vi "15-12-13 UHR-Fleezers Control (host) - 15.2.1UCB Darwin.vi"() -> ()   [LabVIEW 2014] (continued)
                n2143 = Transpose 2D Array(2D array=w3211) -> (transposed array=w3217:u32[][])
                n2144 = Select(t=w3217, s="Flip Y (or X)", f=w3211) -> (s? t:f=w3216:u32[][])
                n2145 = call "DMR_ImageRequestUnlock.vi"("request number IN"=w3232, "driver handle IN"=w3233) -> ("driver handle OUT"=w3238:i32)  [unwired: 1 in, 2 out]
                n2146 = for {
                  tunnel: w3216 -> [w3275] mode=indexing
                  tunnel: [w3274] -> w3214 mode=indexing
                  n2147 = Reverse 1D Array(array=w3275) -> (reversed array=w3274:u32[])
                }
                n2148 = call "DMR_ImageRequestSingle.vi"("request control IN"=0, "driver handle IN"=w3238) -> ("driver handle OUT"=w3236:i32)  [unwired: 3 out]
                n2149 = Transpose 2D Array(2D array=w3214) -> (transposed array=w3215:u32[][])
                n2150 = Select(t=w3215, s="Flip Y (or X)", f=w3214) -> (s? t:f=w3212:u32[][])
                n2151 = Select(t=w3212, s="Flip Image", f=w3211) -> (s? t:f=w3209:u32[][])
                n2152 = case shown="True" "Averaging" {
                  tunnel: w3209 -> [w3286 w3291]
                  tunnel: [w3286 w3290] -> w3223
                  tunnel: w3225 -> [_ w3288]
                  frame False {
                  }
                  frame True {
                    (unwired) 1
                    w3296 = 1
                    n2153 = feedback #2(w3288) -> (w3287:u32[][])
                    n2154 = Add(x=w3291, y=w3287) -> (x+y=w3292:u32[][])
                    n2155 = Select(t=w3288, s="Reset Averaging", f=w3292) -> (s? t:f=w3294:u32[][])
                    n2156 = feedback-in #2(w3294) -> ()
                    n2157 = feedback #3(w3296) -> (w3289:i32)
                    n2158 = Divide(x=w3292, y=w3289) -> (x/y=w3293:dbl[][])
                    n2159 = Increment(x=w3289) -> (x+1=w3297:i32)
                    n2160 = To Unsigned Long Integer(number=w3293) -> (unsigned 32bit integer=w3290:u32[][])
                    n2161 = Select(t=w3296, s="Reset Averaging", f=w3297) -> (s? t:f=w3295:i32)
                    n2162 = feedback-in #3(w3295) -> ()
                  }
                }
                n2163 = case shown="True" "Zoom video window" {
                  tunnel: w3223 -> [_ w3254]
                  tunnel: w3219 -> [_ w3253]
                  frame False {
                  }
                  frame True {
                    n2164 = To Double Precision Float(number=w3254) -> (double precision float=w3251:dbl[][])
                    n2165 = In Range and Coerce(upper limit="Intensity Upper", x=w3251, lower limit="Intensity Lower") -> (coerced(x)=w3250:dbl[][])  [unwired: 1 out]
                    n2166 = Subtract(x="Intensity Upper", y="Intensity Lower") -> (x-y=w3247:dbl)
                    n2167 = Subtract(x=w3250, y="Intensity Lower") -> (x-y=w3248:dbl[][])
                    n2168 = Divide(x=w3248, y=w3247) -> (x/y=w3249:dbl[][])
                    n2169 = Multiply(x=255.0, y=w3249) -> (x*y=w3245:dbl[][])
                    n2170 = To Unsigned Byte Integer(number=w3245) -> (unsigned 8bit integer=w3252:u8[][])
                    n2171 = call "IMAQ ArrayToImage"("Image Pixels (U8)"=w3252, "Image"=w3253) -> ("Image Out"=w3241:T2)  [unwired: 4 in, 5 out]
                    n2172 = First Call?() -> (First Call?: T/F=w3242:bool)
                    n2173 = case shown="True" w3242 {
                      tunnel: w3241 -> [w3255 w3266]
                      frame False {
                        n2174 = flat-sequence {
                          tunnel: w3255 -> [w3261]
                          frame #0 {
                            w3258 = FALSE ("Get/Set Status? (Set)")
                            w3257 = 0 ("Window Number (0...15)")
                            n2175 = call "IMAQ WindSize"("Get/Set Status? (Set)"=w3258, "Window Number"=w3257) -> ("Width & Height out"=→"Window Size":cluster{"Width":i32, "Height":i32})  [unwired: 4 in, 2 out]
                            n2176 = call "IMAQ WindMove"("Window Number (0...15)"=w3257, "Get/Set Status? (Set)"=w3258) -> ("Coordinates (screen)"=→"Window Position":cluster{"X Position":i32, "Y Position":i32})  [unwired: 3 in, 1 out]
                            n2177 = call "IMAQ WindDraw"("Resize to Image Size? (Y)"=FALSE, "Window Number (0...15)"=w3257, "Image"=w3261) -> ()  [unwired: 7 in, 2 out]
                          }
                          frame #1 {
                            n2178 = call "IMAQ WindZoom 2"("Center Point"="Center Point", "Zoom to Fit? (False)"=FALSE, "Zoom Factor"="Zoom Factor") -> ()  [unwired: 5 in, 4 out]
                          }
                        }
                      }
                      frame True {
                        n2179 = flat-sequence {
                          tunnel: w3266 -> [w3269]
                          tunnel: [w3267] -> w3265
                          tunnel: w3265 -> [w3271]
                          frame #0 {
                            w3268 = TRUE ("Resize to Image Size? (Y)")
                            w3267 = 0 ("Window Number (0...15)")
                            n2180 = call "IMAQ WindNonTearing"("Window Number"=w3267, "NonTearing? (True)"=w3268) -> ()  [unwired: 8 in, 2 out]
                            n2181 = call "IMAQ WindDraw"("Resize to Image Size? (Y)"=w3268, "Window Number (0...15)"=w3267, "Image"=w3269) -> ()  [unwired: 7 in, 2 out]
                          }
                          frame #1 {
                            n2182 = call "IMAQ WindSize"("Scrollbars? (N)"=FALSE, "Width & Height"="Initial Window Size", "Window Number"=w3271) -> ()  [unwired: 3 in, 3 out]
                            n2183 = call "IMAQ WindMove"("Window Number (0...15)"=w3271, "Coordinates (screen)"="Initial Window Position") -> ()  [unwired: 3 in, 2 out]
                          }
                        }
                      }
                    }
                  }
                }
                n2184 = To Unsigned Byte Integer(number=w3223) -> (unsigned 8bit integer=w3221:u8[][])
                n2185 = call "IMAQ ArrayToImage"("Image Pixels (U8)"=w3221, "Image"=w3222) -> ("Image Out"=w3220:T2)  [unwired: 4 in, 5 out]
                "Primary Video Display" <- w3220
                n2186 = Not(x="Close Video File") -> (.not. x?=w3207:bool)
                n2187 = And(x="Save Video", y=w3207) -> (x .and. y?=w3204:bool)
                n2188 = case shown="True" "Save Image" {
                  tunnel: w3221 -> [_ w3300]
                  tunnel: w3218 -> [_ w3299]
                  frame False {
                  }
                  frame True {
                    n2189 = call <vilib>:"Flatten Pixmap.vi"("colors"=w3299, "8-bit pixmap"=w3300) -> ("image data"=w3306:T41)  [unwired: 4 in, 5 out]
                    n2190 = call "Create new save file.vi"("Insert"="video_frame_" ("string"), "Ext"=".bmp" ("string"), "Index In"="Image Index") -> ("Path Out"=w3302:path, "Index Out"=w3307:dbl)
                    n2191 = Increment(x=w3307) -> (x+1=w3301:dbl)
                    n2192 = local write "Image Index"(w3301) -> ()
                    n2193 = call <vilib>:"Write BMP File.vi"("image data"=w3306, "path to BMP file"=w3302) -> ()  [unwired: 1 in, 9 out]
                  }
                }
                n2194 = case shown="True" w3204 {
                  tunnel: w3205 -> [w3277 w3282]
                  tunnel: w3220 -> [_ w3281]
                  tunnel: "Close Video File" -> [w3276 _]
                  frame False {
                    n2195 = case shown="True" w3276 {
                      tunnel: w3277 -> [_ w3278]
                      frame False {
                      }
                      frame True {
                        w3279 = FALSE ("Save Video")
                        n2196 = call "IMAQ AVI2 Close"("AVI Refnum"=w3278) -> ()  [unwired: 10 in, 1 out]
                        n2197 = local write "File open?"(w3279) -> ()
                        n2198 = local write "Save Video"(w3279) -> ()
                      }
                    }
                  }
                  frame True {
                    n2199 = local read "File open?"() -> (w3280:bool)
                    n2200 = case shown="True" w3280 {
                      tunnel: w3282 -> [_ w3285]
                      tunnel: w3281 -> [_ w3284]
                      frame False {
                        n2201 = local write "New Video File"(TRUE ("New Video File")) -> ()
                      }
                      frame True {
                        n2202 = call "IMAQ AVI2 Write Frame"("Image"=w3284, "AVI Refnum"=w3285) -> ()  [unwired: 7 in, 3 out]
                      }
                    }
                  }
                }
              }
            }
            n2203 = node-c288(w3167, "Deadline (ms)") -> ()  [unwired: 1 out]
          }
          n2204 = node-c288(w3147) -> ()  [unwired: 1 out]
          n2205 = call "DMR_CloseDevice.vi"("driver handle IN"=w3152) -> ()  [unwired: 1 in, 4 out]
        }
        frame #4 {
          n2206 = call "DMR_Close.vi"() -> ()  [unwired: 1 out]
        }
      }
    }
    frame Enabled {
    }
  }
  n2207 = node-c288(3 ("Processor")) -> (w57:T27)  [unwired: 3 out]
  n2208 = timed-loop "Oscillate Trap/AOM (fishing, conjugate plane alignment)" {
    tunnel: [w3314] -> w62
    timing: w57 -> [_]
    timing-out: [_] -> w56
    tunnel: w15 -> [w3313]
    tunnel: w3 -> [w3312]
    stop <- w3314 stop-if-true
    n2209 = node-c288() -> ()  [unwired: 2 out]
    n2210 = event shown="[2] \"Start assembly line\": Value Change" {
      selector: _ -> [_ _ _ _]
      dyn-events: _ -> [_ _ _ _]
      timeout: _ -> [_ _ _ _]
      tunnel: [FALSE ("Stop All") _ _ w3985] -> w3314
      tunnel: w3313 -> [w3317 _ _ _]
      tunnel: w3312 -> [_ _ w3922 _]
      event "Oscillate Set 1", "Fish for Tether": Value Change {
        n2211 = event-data() -> ()  [unwired: 6 out]
        n2212 = local read "Oscillate Set 1"() -> (w3321:bool)
        n2213 = Or(x=w3321, y="Fish for Tether") -> (x .or. y?=w3319:bool)
        n2214 = case shown="True" w3319 {
          tunnel: "Fish for Tether" -> [_ w3324]
          tunnel: w3317 -> [_ w3322]
          frame False {
          }
          frame True {
            n2215 = case shown="True" w3324 {
              selector: w3324 -> [w3327 w3333]
              tunnel: [w3327 w3333] -> w3323
              frame False {
              }
              frame True {
                n2216 = local write "Scan axis 2"(TRUE) -> ()
                n2217 = local write "Tether"(FALSE ("Tether")) -> ()
                n2218 = local read "Flow ON during cal?"() -> (w3328:bool)
                n2219 = property on="Trap Delta (MHz)" class="DigNum (strict)"("Val(Sgnl)"="Furthest Delta (MHz)") -> ()  [unwired: 2 in, 2 out]
                n2220 = Or(x="Flow ON during \nfishing?", y=w3328) -> (x .or. y?=w3329:bool)
                n2221 = Wait (ms)(milliseconds to wait=u32 500) -> ()  [unwired: 1 out]
                n2222 = property on="Sample Channel\nFlow" class="Bool (strict)"("Val(Sgnl)"=w3329) -> ()  [unwired: 2 in, 2 out]
              }
            }
            n2223 = node-c288() -> (w3326:T27)  [unwired: 1 in, 3 out]
            n2224 = timed-loop "Oscillate AOD" {
              timing: w3326 -> [_]
              timing-out: [_] -> w3325
              tunnel: w3323 -> [w3337]
              tunnel: w3322 -> [w3336]
              i -> [w3345]
              stop <- w3343 stop-if-true
              n2225 = node-c288() -> (w3344:i64)  [unwired: 1 out]
              n2226 = flat-sequence {
                tunnel: w3345 -> [w3372]
                tunnel: w3344 -> [w3371]
                tunnel: w3337 -> [w3355]
                tunnel: [w3355] -> w3342
                tunnel: [w3354] -> w3341
                tunnel: [w3353] -> w3340
                tunnel: [w3350] -> w3338
                tunnel: w3336 -> [w3346]
                tunnel: w3342 -> [w3419]
                tunnel: w3341 -> [w3417]
                tunnel: w3340 -> [w3416]
                tunnel: [w3415] -> w3339
                tunnel: w3338 -> [w3414]
                tunnel: [w3491] -> w3343
                tunnel: w3339 -> [w3490]
                frame #0 {
                  # "w (rad/s)"
                  # "t (s)"
                  n2227 = Divide(x=w3371, y=i64 1000) -> (x/y=w3347:dbl)
                  n2228 = local read "BD 1 Frequency 2 (MHz)"() -> (w3349:dbl)
                  n2229 = Multiply(x="Osc. freq. (Hz)", y=6.283185307179586) -> (x*y=w3369:dbl)
                  n2230 = Multiply(x=w3347, y=w3372) -> (x*y=w3368:dbl)
                  n2231 = Multiply(x=w3369, y=w3368) -> (x*y=w3352:dbl)
                  n2232 = local read "BD 1 Frequency 1 (MHz)"() -> (w3357:dbl)
                  n2233 = case shown="True" w3355 {
                    tunnel: w3352 -> [w3378 w3397]
                    tunnel: w3357 -> [_ w3405]
                    tunnel: w3349 -> [_ w3406]
                    tunnel: [w3375 w3401] -> w3348
                    tunnel: [FALSE w3379] -> w3353
                    tunnel: [0.0 w3393] -> w3350
                    frame False {
                      n2234 = Sine(x=w3378) -> (sin(x)=w3376:dbl)
                      n2235 = Multiply(x=w3376, y="Osc. amp. (MHz)") -> (x*y=w3375:dbl)
                    }
                    frame True {
                      # "trap position goes from 0 to 1 (0 is when it is furthest away, 1 is when closest)\nso we want to test for tether only when farther away, or x < 1"
                      # "quit if taking too long"
                      # "oscillate the trap"
                      # "Test for tether"
                      n2236 = local read "Vec Mean of T1 T2"() -> (w3382:dbl[])
                      "Trigger Signal" <- w3382
                      n2237 = Cosine(x=w3397) -> (cos(x)=w3409:dbl)
                      n2238 = Subtract(x=w3406, y=w3405) -> (x-y=w3404:dbl)
                      n2239 = Decrement(x=w3409) -> (x-1=w3408:dbl)
                      n2240 = Subtract(x=w3404, y="Closest Delta (MHz)") -> (x-y=w3402:dbl)
                      n2241 = Divide(x=w3408, y=-2.0) -> (x/y=w3392:dbl)
                      n2242 = Greater?(x=w3382, y="Stop F (pN)") -> (0:w3399:bool[])
                      n2243 = Multiply(x=w3392, y=w3402) -> (x*y=w3401:dbl)
                      n2244 = Less?(x=w3392, y="Fish mask thresh") -> (x < y?=w3391:bool)
                      n2245 = Boolean To (0,1)(Boolean=w3391) -> (0, 1=w3389:i16)
                      n2246 = Multiply(x=w3389, y=w3382) -> (x*y=w3388:dbl[])
                      n2247 = Divide(x=w3397, y=6.283185307179586) -> (x/y=w3396:dbl)
                      n2248 = Round Toward +Infinity(x=w3396) -> (ceil(x): smallest int >= x=w3393:dbl)
                      "Attempts" <- w3393
                      n2249 = Greater?(x=w3388, y="Stop F (pN) (mask)") -> (0:w3386:bool[])
                      n2250 = Or Array Elements(Boolean array=w3399) -> (logical OR=w3384:bool)
                      n2251 = Or Array Elements(Boolean array=w3386) -> (logical OR=w3383:bool)
                      n2252 = Greater?(x=w3393, y="Attempt Limit") -> (0:w3395:bool)
                      n2253 = case shown="True" w3395 {
                        frame False {
                        }
                        frame True {
                          n2254 = local write "Fish for Tether"(FALSE ("Fish for Tether")) -> ()
                          n2255 = call <vilib>:"Beep.vi"() -> ()  [unwired: 3 in, 9 out]
                          n2256 = local read "Messages"() -> (w3411:string)
                          n2257 = call "Update messages.vi"("Message to add"="Tether fishing timeout." ("Messages"), "Old message string"=w3411) -> ("New message string"=→"Messages":string)
                        }
                      }
                      n2258 = Select(t=w3384, s="Normal (on) or masked test (off)", f=w3383) -> (s? t:f=w3381:bool)
                      n2259 = And(x="Stop Fishing When Tether", y=w3381) -> (x .and. y?=w3379:bool)
                    }
                  }
                  n2260 = local read "BD 2 Frequency 1 (MHz)"() -> (w3356:dbl)
                  n2261 = Select(t=w3357, s="Scan axis 2", f=w3356) -> (s? t:f=w3360:dbl)
                  n2262 = Add(x=w3348, y=w3360) -> (x+y=w3354:dbl)
                  n2263 = Select(t=w3354, s="Scan axis 2", f=w3357) -> (s? t:f=w3363:dbl)
                  n2264 = Select(t=w3356, s="Scan axis 2", f=w3354) -> (s? t:f=w3362:dbl)
                  n2265 = local read "BD 2 Frequency 2 (MHz)"() -> (w3365:dbl)
                  n2266 = local read "BD 2 Frequency 3 (MHz)"() -> (w3364:dbl)
                  n2267 = local read "Y RF Frequency Limits (MHz)"() -> (w3358:T18)
                  n2268 = local read "X RF Frequency Limits (MHz)"() -> (w3359:T18)
                  n2269 = local read "BD 1 Frequency 3 (MHz)"() -> (w3366:dbl)
                  n2270 = call "set RF board frequency - interlace.vi"("Board 2 Frequency Limits"=w3358, "Board 1 Frequency Limits"=w3359, "FPGA VI Reference In"=w3346, "Board 2 Frequency 3 (MHz)"=w3364, "Board 1 Frequency 3 (MHz)"=w3366, "Board 2 Frequency 2 (MHz)"=w3365, "Board 2 Frequency 1 (MHz)"=w3362, "Board 1 Frequency 2 (MHz)"=w3349, "Board 1 Frequency 1  (MHz)"=w3363) -> ()  [unwired: 1 in, 2 out]
                }
                frame #1 {
                  n2271 = And(x=w3419, y=w3416) -> (x .and. y?=w3418:bool)
                  n2272 = case "Only if were fishing and now formed tether" shown="True" w3418 {
                    tunnel: w3417 -> [w3421 w3436]
                    tunnel: [w3420 w3435] -> w3415
                    tunnel: w3414 -> [_ w3431]
                    frame False {
                      n2273 = local read "Fish for Tether"() -> (w3420:bool)
                      n2274 = case shown="False" w3420 {
                        tunnel: w3421 -> [w3422 _]
                        frame False {
                          n2275 = property on="BD 1 Frequency 1 (MHz)" class="DigNum (strict)"("Val(Sgnl)"=w3422) -> ()  [unwired: 2 in, 2 out]
                        }
                        frame True {
                        }
                      }
                    }
                    frame True {
                      w3435 = FALSE ("Fish for Tether")
                      n2276 = call <vilib>:"Beep.vi"() -> ()  [unwired: 3 in, 9 out]
                      n2277 = Number To Decimal String(number=w3431, width (-)=i16 1) -> (decimal integer string=w3429:string)
                      n2278 = Concatenate Strings("Formed tether in ", w3429, " attempt(s)." ("string")) -> (w3426:string)
                      n2279 = local read "Messages"() -> (w3433:string)
                      n2280 = local write "Fish for Tether"(w3435) -> ()
                      n2281 = call "Update messages.vi"("Message to add"=w3426, "Old message string"=w3433) -> ("New message string"=w3432:string)
                      n2282 = local write "Messages"(w3432) -> ()
                      n2283 = Get Date/Time In Seconds() -> (seconds since 1Jan1904=→"Time tether formed":timestamp)
                      n2284 = local read "Flow ON during cal?"() -> (w3423:bool)
                      n2285 = property on="Sample Channel\nFlow" class="Bool (strict)"("Val(Sgnl)"=w3423) -> (error out=w3424:errorcluster)  [unwired: 2 in, 1 out]
                      n2286 = case shown="\"2\", \"3\", \"4\", \"5\", \"6\"" "Then..." {
                        selector: "Then..." -> [_ w3439]
                        tunnel: w3436 -> [w3438 _]
                        tunnel: w3424 -> [_ _]
                        frame "1", Default {
                          n2287 = property on="BD 1 Frequency 1 (MHz)" class="DigNum (strict)"("Val(Sgnl)"=w3438) -> ()  [unwired: 2 in, 2 out]
                        }
                        frame "2", "3", "4", "5", "6" {
                          n2288 = flat-sequence {
                            tunnel: w3439 -> [w3441]
                            frame #0 {
                              n2289 = property on="Trap Delta (MHz)" class="DigNum (strict)"("Val(Sgnl)"="Move to Delta 1 (MHz)") -> ()  [unwired: 2 in, 2 out]
                            }
                            frame #1 {
                              n2290 = case shown="\"5\", \"6\"" w3441 {
                                selector: w3441 -> [w3444 w3454 _]
                                frame "3", "4" {
                                n2291 = flat-sequence {
                                tunnel: w3444 -> [w3445]
                                tunnel: [w3445] -> w3442
                                tunnel: [w3447] -> w3443
                                tunnel: w3442 -> [w3447]
                                tunnel: w3443 -> [w3451]
                                frame #0 {
                                n2292 = property on="Green Laser ON" class="Bool (strict)"("Val(Sgnl)"=TRUE ("Value (Signaling)")) -> ()  [unwired: 2 in, 2 out]
                                }
                                frame #1 {
                                n2293 = Multiply(x="Wait Before Save (s)", y=u32 1000 ("x")) -> (x*y=w3449:u32)
                                n2294 = Wait (ms)(milliseconds to wait=w3449) -> ()  [unwired: 1 out]
                                }
                                frame #2 {
                                n2295 = property on="Start Saving" class="Bool (strict)"("Value"=TRUE ("Start Saving")) -> ()  [unwired: 2 in, 2 out]
                                n2296 = case shown="\"4\"" w3451 {
                                frame Default {
                                }
                                frame "4" {
                                n2297 = property on="Fl. Triggered..." class="Bool (strict)"("Val(Sgnl)"=TRUE ("Value (Signaling)")) -> ()  [unwired: 2 in, 2 out]
                                }
                                }
                                }
                                }
                                }
                                frame "5", "6" {
                                n2298 = stacked-sequence {
                                tunnel: w3454 -> [_ _ _ _ _ _ w3466]
                                frame #0 {
                                n2299 = Replace Array Subset(array=u32[] [0] ("Index Values"), new element="Raster Set Upon Tether", index=0) -> (w3455:u32[])
                                n2300 = property on="Saved AOD Raster Scan Parameter Sets" class="Arr (strict)"("Index Values"=w3455) -> ()  [unwired: 2 in, 2 out]
                                }
                                frame #1 {
                                n2301 = Wait (ms)(milliseconds to wait=u32 500) -> ()  [unwired: 1 out]
                                }
                                frame #2 {
                                n2302 = property on="Load parameters" class="Bool (strict)"("Val(Sgnl)"=TRUE ("Value (Signaling)")) -> ()  [unwired: 2 in, 2 out]
                                n2303 = case shown="True" "Green ON During Raster" {
                                frame False {
                                }
                                frame True {
                                n2304 = property on="Green Laser ON" class="Bool (strict)"("Val(Sgnl)"=TRUE ("Value (Signaling)")) -> ()  [unwired: 2 in, 2 out]
                                }
                                }
                                }
                                frame #3 {
                                n2305 = Wait (ms)(milliseconds to wait=u32 500) -> ()  [unwired: 1 out]
                                }
                                frame #4 {
                                n2306 = property on="Trap Raster Scan" class="Bool (strict)"("Val(Sgnl)"=TRUE ("Value (Signaling)")) -> ()  [unwired: 2 in, 2 out]
                                }
                                frame #5 {
                                n2307 = Wait (ms)(milliseconds to wait=u32 2000) -> ()  [unwired: 1 out]
                                }
                                frame #6 {
                                n2308 = flat-sequence {
                                tunnel: w3466 -> [w3473]
                                frame #0 {
                                n2309 = while {
                                stop <- w3469 stop-if-true
                                n2310 = local read "Raster Scanning..."() -> (w3468:bool)
                                n2311 = local read "Saving..."() -> (w3471:bool)
                                n2312 = Wait (ms)(milliseconds to wait=u32 100) -> ()  [unwired: 1 out]
                                n2313 = Not(x=w3471) -> (.not. x?=w3470:bool)
                                n2314 = Not(x=w3468) -> (.not. x?=w3467:bool)
                                n2315 = And(x=w3470, y=w3467) -> (x .and. y?=w3469:bool)
                                }
                                }
                                frame #1 {
                                n2316 = local read "Tether"() -> (w3474:bool)
                                n2317 = case shown="True" w3474 {
                                tunnel: w3473 -> [_ w3476]
                                frame False {
                                n2318 = property on="Fish for Tether" class="Bool (strict)"("Val(Sgnl)"="Fish again after \nraster break?") -> ()  [unwired: 2 in, 2 out]
                                }
                                frame True {
                                n2319 = stacked-sequence {
                                tunnel: w3476 -> [_ w3480 _ _]
                                frame #0 {
                                n2320 = property on="Trap Delta (MHz)" class="DigNum (strict)"("Val(Sgnl)"="Move to Delta 2 (MHz)") -> ()  [unwired: 2 in, 2 out]
                                n2321 = case shown="True" "Flow ON after\ntether testing?" {
                                frame False {
                                }
                                frame True {
                                n2322 = property on="Sample Channel\nFlow" class="Bool (strict)"("Val(Sgnl)"=TRUE ("Value (Signaling)")) -> ()  [unwired: 2 in, 2 out]
                                }
                                }
                                }
                                frame #1 {
                                n2323 = flat-sequence {
                                tunnel: w3480 -> [w3482]
                                frame #0 {
                                n2324 = Wait (ms)(milliseconds to wait=u32 500) -> ()  [unwired: 1 out]
                                }
                                frame #1 {
                                n2325 = case shown="\"6\"" w3482 {
                                frame Default {
                                }
                                frame "6" {
                                n2326 = property on="Green Laser ON" class="Bool (strict)"("Val(Sgnl)"=TRUE ("Green Laser ON/Interlacing")) -> ()  [unwired: 2 in, 2 out]
                                }
                                }
                                }
                                frame #2 {
                                n2327 = Wait (ms)(milliseconds to wait=u32 500) -> ()  [unwired: 1 out]
                                }
                                frame #3 {
                                n2328 = local write "Start Saving"("Save at end (5, 6)") -> ()
                                }
                                }
                                }
                                frame #2 {
                                n2329 = local read "Bead Sep. Int. Time (s)"() -> (w3488:dbl)
                                n2330 = Multiply(x=w3488, y=1000.0) -> (x*y=w3487:dbl)
                                n2331 = Wait (ms)(milliseconds to wait=w3487) -> ()  [unwired: 1 out]
                                }
                                frame #3 {
                                n2332 = property on="Remove Offset" class="Bool (strict)"("Val(Sgnl)"=TRUE ("Value (Signaling)")) -> ()  [unwired: 2 in, 2 out]
                                }
                                }
                                }
                                }
                                }
                                }
                                }
                                }
                                }
                                frame "2", Default {
                                }
                              }
                            }
                          }
                        }
                      }
                      "Tether" <- "Tether Alarm?"
                    }
                  }
                }
                frame #2 {
                  n2333 = local read "Oscillate Set 1"() -> (w3495:bool)
                  n2334 = local read "Stop All"() -> (w3493:bool)
                  n2335 = Or(x=w3495, y=w3490) -> (x .or. y?=w3492:bool)
                  n2336 = Not(x=w3492) -> (.not. x?=w3494:bool)
                  n2337 = Compound Arithmetic op=OR(w3493, w3494) -> (w3491:bool)
                }
              }
              n2338 = node-c288() -> ()  [unwired: 2 out]
            }
            n2339 = node-c288(w3325) -> ()  [unwired: 1 out]
          }
        }
      }
      event "Fl. Triggered...": Value Change {
        n2340 = event-data() -> ()  [unwired: 7 out]
        n2341 = case shown="True" "Fl. Triggered..." {
          frame False {
          }
          frame True {
            n2342 = node-c288() -> (w3506:T27)  [unwired: 4 out]
            n2343 = timed-loop {
              timing: w3506 -> [_]
              timing-out: [_] -> w3505
              tunnel: "Action" -> [w3514]
              shift-right: [w3511] -> _
              shift-left: u8 255 -> [w3513]
              shift-right: [w3508] -> _
              shift-left: 255 -> [w3510]
              stop <- w3507 stop-if-true
              # "Reset confocal spot"
              n2344 = node-c288() -> ()  [unwired: 2 out]
              n2345 = flat-sequence {
                tunnel: w3514 -> [w3534]
                tunnel: w3513 -> [w3533]
                tunnel: [w3532] -> w3512
                tunnel: w3510 -> [w3519]
                tunnel: [w3518] -> w3509
                tunnel: [w3913] -> w3507
                tunnel: w3512 -> [w3912]
                tunnel: [w3912] -> w3511
                tunnel: [w3911] -> w3508
                tunnel: w3509 -> [w3911]
                frame #0 {
                  n2346 = local read "Delta Fl. 2"() -> (w3531:dbl)
                  n2347 = local read "Delta Fl. 1"() -> (w3526:dbl)
                  n2348 = Multiply(x="Fl. Delta Thresh. (kHz)", y=1000.0) -> (x*y=w3521:dbl)
                  n2349 = Select(t=w3526, s="APD to Watch", f=w3531) -> (s? t:f=w3522:dbl)
                  n2350 = Greater?(x=w3522, y=w3521) -> (0:w3527:bool)
                  n2351 = Or(x="Force Yank", y=w3527) -> (x .or. y?=w3525:bool)
                  n2352 = And(x=w3525, y="Yank when?") -> (x .and. y?=w3523:bool)
                  n2353 = case shown="False" w3523 {
                    tunnel: w3534 -> [w3537 w3738]
                    tunnel: w3533 -> [w3539 w3734]
                    tunnel: [w3539 w3732] -> w3532
                    tunnel: w3522 -> [w3545 _]
                    tunnel: w3521 -> [w3544 _]
                    tunnel: "Force Yank" -> [w3542 _]
                    tunnel: w3519 -> [w3541 w3731]
                    tunnel: [w3540 w3731] -> w3518
                    frame False {
                      n2354 = Negate(x=w3544) -> (-x=w3536:dbl)
                      n2355 = local write "Fl. High"(TRUE ("Fl. High")) -> ()
                      n2356 = Less?(x=w3545, y=w3536) -> (x < y?=w3543:bool)
                      n2357 = Or(x=w3542, y=w3543) -> (x .or. y?=w3538:bool)
                      n2358 = case shown="True" w3538 {
                        tunnel: w3541 -> [w3546 w3556]
                        tunnel: [w3546 w3555] -> w3540
                        tunnel: w3537 -> [_ w3554]
                        frame False {
                        }
                        frame True {
                          n2359 = flat-sequence {
                            tunnel: w3556 -> [w3562]
                            tunnel: w3554 -> [w3559]
                            tunnel: [w3561] -> w3553
                            tunnel: [w3560] -> w3552
                            tunnel: [w3559] -> w3551
                            tunnel: w3550 -> [w3558]
                            tunnel: [w3558] -> w3549
                            tunnel: w3548 -> [w3557]
                            tunnel: [w3557] -> w3547
                            tunnel: [w3633] -> w3555
                            tunnel: w3553 -> [w3633]
                            tunnel: w3552 -> [w3632]
                            tunnel: w3551 -> [w3631]
                            tunnel: w3549 -> [w3630]
                            tunnel: w3547 -> [w3629]
                            frame #0 {
                              n2360 = call <vilib>:"Beep.vi"() -> ()  [unwired: 12 in]
                              n2361 = local write "Waiting"(FALSE ("Waiting")) -> ()
                              n2362 = Increment(x=w3562) -> (x+1=w3561:i32)
                              n2363 = case shown="\"Image\"" w3559 {
                                tunnel: w3561 -> [_ w3567 _]
                                frame "Alarm", Default {
                                }
                                frame "Yank" {
                                n2364 = flat-sequence {
                                tunnel: w3567 -> [w3570]
                                tunnel: [w3569] -> w3566
                                tunnel: [w3568] -> w3565
                                tunnel: w3566 -> [w3580]
                                tunnel: w3565 -> [w3581]
                                frame #0 {
                                n2365 = local read "Yank Delay (s)"() -> (w3573:dbl)
                                n2366 = local read "N Array El"() -> (w3568:u8)
                                n2367 = Quotient & Remainder(x=w3570, y=w3568) -> (x-y*floor(x/y)=w3569:i32)  [unwired: 1 out]
                                n2368 = Multiply(x=w3573, y=1000.0) -> (x*y=w3571:dbl)
                                n2369 = Wait (ms)(milliseconds to wait=w3571) -> ()  [unwired: 1 out]
                                }
                                frame #1 {
                                n2370 = local read "Yank to which?"() -> (w3575:bool)
                                n2371 = local read "Random Choice"() -> (w3585:bool)
                                n2372 = local read "Yank to Trap Delta (MHz)"() -> (w3578:dbl[])
                                n2373 = local read "Yank to SP"() -> (w3579:dbl[])
                                n2374 = Random Number (0-1)() -> (number: 0 to 1=w3584:dbl)
                                n2375 = Multiply(x=w3581, y=w3584) -> (x*y=w3583:dbl)
                                n2376 = Round Toward -Infinity(1:w3583) -> (0:w3582:dbl)
                                n2377 = Select(t=w3582, s=w3585, f=w3580) -> (s? t:f=w3576:dbl)
                                n2378 = Select(t=w3578, s=w3575, f=w3579) -> (s? t:f=w3577:dbl[])
                                n2379 = Index Array(array=w3577, index=w3576) -> (element=w3574:dbl)
                                n2380 = case shown="True" w3575 {
                                tunnel: w3574 -> [w3586 w3613]
                                frame False {
                                n2381 = flat-sequence {
                                tunnel: w3586 -> [w3587]
                                frame #0 {
                                n2382 = property on="Trap Pos FB SP" class="DigNum (strict)"("Val(Sgnl)"=w3587) -> ()  [unwired: 2 in, 2 out]
                                }
                                frame #1 {
                                n2383 = Wait (ms)(milliseconds to wait=u32 700) -> ()  [unwired: 1 out]
                                }
                                frame #2 {
                                n2384 = local read "Action (%)"() -> (w3592:dbl)
                                n2385 = Absolute Value(x=w3592) -> (abs(x)=w3591:dbl)
                                n2386 = Greater?(x=w3591, y=70.0) -> (0:w3589:bool)
                                n2387 = property on="Remove Action Offset" class="Bool (strict)"("Val(Sgnl)"=w3589) -> ()  [unwired: 2 in, 2 out]
                                }
                                frame #3 {
                                n2388 = for {
                                N: 4 -> [_]
                                n2389 = flat-sequence {
                                frame #0 {
                                n2390 = Wait (ms)(milliseconds to wait=u32 500) -> ()  [unwired: 1 out]
                                }
                                frame #1 {
                                n2391 = local read "Action (%)"() -> (w3598:dbl)
                                n2392 = Absolute Value(x=w3598) -> (abs(x)=w3597:dbl)
                                n2393 = Greater?(x=w3597, y=70.0) -> (0:w3595:bool)
                                n2394 = property on="Remove Action Offset" class="Bool (strict)"("Val(Sgnl)"=w3595) -> ()  [unwired: 2 in, 2 out]
                                }
                                }
                                }
                                }
                                frame #4 {
                                n2395 = Wait (ms)(milliseconds to wait=u32 500) -> ()  [unwired: 1 out]
                                }
                                frame #5 {
                                n2396 = local read "Mean"() -> (w3606:dbl)
                                n2397 = Greater?(x=w3606, y=11.0) -> (0:w3600:bool)
                                n2398 = Not(x=w3600) -> (.not. x?=w3601:bool)
                                n2399 = And(x=w3601, y="Shift confocal") -> (x .and. y?=w3603:bool)
                                n2400 = And(x=w3600, y="Shift confocal") -> (x .and. y?=w3604:bool)
                                n2401 = case shown="True" w3604 {
                                frame False {
                                }
                                frame True {
                                n2402 = local read "Confocal Y 2 (V)"() -> (w3610:dbl)
                                n2403 = local read "Confocal X 2 (V)"() -> (w3609:dbl)
                                n2404 = property on="AO1" class="Slide (strict)"("Val(Sgnl)"=w3610) -> ()  [unwired: 2 in, 2 out]
                                n2405 = property on="AO2" class="Slide (strict)"("Val(Sgnl)"=w3609) -> ()  [unwired: 2 in, 2 out]
                                }
                                }
                                n2406 = case shown="True" w3603 {
                                frame False {
                                }
                                frame True {
                                n2407 = local read "Confocal Y 1 (V)"() -> (w3608:dbl)
                                n2408 = local read "Confocal X 1 (V)"() -> (w3607:dbl)
                                n2409 = property on="AO1" class="Slide (strict)"("Val(Sgnl)"=w3608) -> ()  [unwired: 2 in, 2 out]
                                n2410 = property on="AO2" class="Slide (strict)"("Val(Sgnl)"=w3607) -> ()  [unwired: 2 in, 2 out]
                                }
                                }
                                }
                                frame #6 {
                                n2411 = Wait (ms)(milliseconds to wait=u32 1500) -> ()  [unwired: 1 out]
                                }
                                frame #7 {
                                n2412 = property on="Rem fb disp offset" class="Bool (strict)"("Val(Sgnl)"=TRUE ("Value (Signaling)")) -> ()  [unwired: 2 in, 2 out]
                                }
                                }
                                }
                                frame True {
                                n2413 = flat-sequence {
                                tunnel: w3613 -> [w3614]
                                frame #0 {
                                n2414 = property on="Trap Delta (MHz)" class="DigNum (strict)"("Val(Sgnl)"=w3614) -> ()  [unwired: 2 in, 2 out]
                                }
                                frame #1 {
                                n2415 = Wait (ms)(milliseconds to wait=u32 500) -> ()  [unwired: 1 out]
                                }
                                frame #2 {
                                n2416 = local read "Shift confocal"() -> (w3620:bool)
                                n2417 = local read "Mean"() -> (w3622:dbl)
                                n2418 = Greater?(x=w3622, y=11.0) -> (0:w3619:bool)
                                n2419 = Not(x=w3619) -> (.not. x?=w3618:bool)
                                n2420 = And(x=w3618, y=w3620) -> (x .and. y?=w3616:bool)
                                n2421 = And(x=w3619, y=w3620) -> (x .and. y?=w3617:bool)
                                n2422 = case shown="True" w3617 {
                                frame False {
                                }
                                frame True {
                                n2423 = local read "Confocal Y 2 (V)"() -> (w3626:dbl)
                                n2424 = local read "Confocal X 2 (V)"() -> (w3625:dbl)
                                n2425 = property on="AO2" class="Slide (strict)"("Val(Sgnl)"=w3625) -> ()  [unwired: 2 in, 2 out]
                                n2426 = property on="AO1" class="Slide (strict)"("Val(Sgnl)"=w3626) -> ()  [unwired: 2 in, 2 out]
                                }
                                }
                                n2427 = case shown="True" w3616 {
                                frame False {
                                }
                                frame True {
                                n2428 = local read "Confocal X 1 (V)"() -> (w3623:dbl)
                                n2429 = local read "Confocal Y 1 (V)"() -> (w3624:dbl)
                                n2430 = property on="AO2" class="Slide (strict)"("Val(Sgnl)"=w3623) -> ()  [unwired: 2 in, 2 out]
                                n2431 = property on="AO1" class="Slide (strict)"("Val(Sgnl)"=w3624) -> ()  [unwired: 2 in, 2 out]
                                }
                                }
                                }
                                }
                                }
                                }
                                }
                                }
                                }
                                frame "Image" {
                                n2432 = property on="Confocal Image" class="Bool (strict)"("Val(Sgnl)"=TRUE ("Value (Signaling)")) -> ()  [unwired: 2 in, 2 out]
                                }
                              }
                              n2433 = local write "Fl. High"(FALSE ("Fl. High")) -> ()
                              n2434 = local read "Time (s)"() -> (w3560:dbl)
                            }
                            frame #1 {
                              n2435 = case shown="True" "Auto F Reset" {
                                tunnel: w3632 -> [_ w3637]
                                tunnel: w3631 -> [_ w3636]
                                tunnel: w3630 -> [_ w3635]
                                tunnel: w3629 -> [_ w3634]
                                frame False {
                                }
                                frame True {
                                n2436 = node-c288() -> (w3639:T27)  [unwired: 4 in]
                                n2437 = timed-loop {
                                timing: w3639 -> [_]
                                timing-out: [_] -> w3638
                                tunnel: w3637 -> [w3644]
                                tunnel: w3636 -> [w3643]
                                tunnel: w3635 -> [w3642]
                                tunnel: w3634 -> [w3641]
                                stop <- w3640 stop-if-true
                                n2438 = node-c288() -> ()  [unwired: 1 in, 1 out]
                                n2439 = local read "Fl. Delta Thresh. (kHz)"() -> (w3653:dbl)
                                n2440 = local read "APD to Watch"() -> (w3654:bool)
                                n2441 = local read "Delta Fl. 1"() -> (w3655:dbl)
                                n2442 = local read "Delta Fl. 2"() -> (w3656:dbl)
                                n2443 = local read "Fl. Triggered..."() -> (w3647:bool)
                                n2444 = local read "Stop All"() -> (w3648:bool)
                                n2445 = local read "Reset Force"() -> (w3646:bool)
                                n2446 = Multiply(x=w3653, y=1000.0) -> (x*y=w3651:dbl)
                                n2447 = Select(t=w3655, s=w3654, f=w3656) -> (s? t:f=w3650:dbl)
                                n2448 = Not(x=w3647) -> (.not. x?=w3645:bool)
                                n2449 = Greater?(x=w3650, y=w3651) -> (0:w3649:bool)
                                n2450 = Compound Arithmetic op=OR(w3649, w3648, w3645, w3646) -> (w3640:bool)
                                n2451 = case shown="True" w3640 {
                                tunnel: w3644 -> [_ w3660]
                                tunnel: w3643 -> [_ w3664]
                                tunnel: w3642 -> [_ w3663]
                                tunnel: w3641 -> [_ w3662]
                                frame False {
                                }
                                frame True {
                                n2452 = case shown="\"Yank\"" w3664 {
                                tunnel: w3663 -> [_ w3674]
                                tunnel: w3662 -> [_ w3672]
                                frame "Image", Default {
                                }
                                frame "Yank" {
                                n2453 = flat-sequence {
                                tunnel: [w3677] -> w3675
                                tunnel: w3674 -> [w3677]
                                tunnel: [w3676] -> w3673
                                tunnel: w3672 -> [w3676]
                                tunnel: w3675 -> [w3683]
                                tunnel: w3673 -> [w3681]
                                frame #0 {
                                n2454 = local read "Yank Delay (s)"() -> (w3680:dbl)
                                n2455 = Multiply(x=w3680, y=1000.0) -> (x*y=w3678:dbl)
                                n2456 = Wait (ms)(milliseconds to wait=w3678) -> ()  [unwired: 1 out]
                                }
                                frame #1 {
                                n2457 = local read "Yank to which?"() -> (w3682:bool)
                                n2458 = case shown="False" w3682 {
                                tunnel: w3683 -> [_ w3711]
                                tunnel: w3681 -> [w3684 _]
                                frame False {
                                n2459 = flat-sequence {
                                tunnel: w3684 -> [w3685]
                                frame #0 {
                                n2460 = property on="Trap Pos FB SP" class="DigNum (strict)"("Val(Sgnl)"=w3685) -> ()  [unwired: 2 in, 2 out]
                                }
                                frame #1 {
                                n2461 = Wait (ms)(milliseconds to wait=u32 700) -> ()  [unwired: 1 out]
                                }
                                frame #2 {
                                n2462 = local read "Action (%)"() -> (w3690:dbl)
                                n2463 = Absolute Value(x=w3690) -> (abs(x)=w3689:dbl)
                                n2464 = Greater?(x=w3689, y=70.0) -> (0:w3687:bool)
                                n2465 = property on="Remove Action Offset" class="Bool (strict)"("Val(Sgnl)"=w3687) -> ()  [unwired: 2 in, 2 out]
                                }
                                frame #3 {
                                n2466 = for {
                                N: 4 -> [_]
                                n2467 = flat-sequence {
                                frame #0 {
                                n2468 = Wait (ms)(milliseconds to wait=u32 500) -> ()  [unwired: 1 out]
                                }
                                frame #1 {
                                n2469 = local read "Action (%)"() -> (w3696:dbl)
                                n2470 = Absolute Value(x=w3696) -> (abs(x)=w3695:dbl)
                                n2471 = Greater?(x=w3695, y=70.0) -> (0:w3693:bool)
                                n2472 = property on="Remove Action Offset" class="Bool (strict)"("Val(Sgnl)"=w3693) -> ()  [unwired: 2 in, 2 out]
                                }
                                }
                                }
                                }
                                frame #4 {
                                n2473 = Wait (ms)(milliseconds to wait=u32 500) -> ()  [unwired: 1 out]
                                }
                                frame #5 {
                                n2474 = local read "Shift confocal"() -> (w3701:bool)
                                n2475 = local read "Mean"() -> (w3704:dbl)
                                n2476 = Greater?(x=w3704, y=11.0) -> (0:w3700:bool)
                                n2477 = Not(x=w3700) -> (.not. x?=w3699:bool)
                                n2478 = And(x=w3700, y=w3701) -> (x .and. y?=w3702:bool)
                                n2479 = And(x=w3699, y=w3701) -> (x .and. y?=w3698:bool)
                                n2480 = case shown="True" w3702 {
                                frame False {
                                }
                                frame True {
                                n2481 = local read "Confocal X 2 (V)"() -> (w3707:dbl)
                                n2482 = local read "Confocal Y 2 (V)"() -> (w3708:dbl)
                                n2483 = property on="AO2" class="Slide (strict)"("Val(Sgnl)"=w3707) -> ()  [unwired: 2 in, 2 out]
                                n2484 = property on="AO1" class="Slide (strict)"("Val(Sgnl)"=w3708) -> ()  [unwired: 2 in, 2 out]
                                }
                                }
                                n2485 = case shown="True" w3698 {
                                frame False {
                                }
                                frame True {
                                n2486 = local read "Confocal Y 1 (V)"() -> (w3706:dbl)
                                n2487 = local read "Confocal X 1 (V)"() -> (w3705:dbl)
                                n2488 = property on="AO1" class="Slide (strict)"("Val(Sgnl)"=w3706) -> ()  [unwired: 2 in, 2 out]
                                n2489 = property on="AO2" class="Slide (strict)"("Val(Sgnl)"=w3705) -> ()  [unwired: 2 in, 2 out]
                                }
                                }
                                }
                                frame #6 {
                                n2490 = Wait (ms)(milliseconds to wait=u32 1500) -> ()  [unwired: 1 out]
                                }
                                frame #7 {
                                n2491 = property on="Rem fb disp offset" class="Bool (strict)"("Val(Sgnl)"=TRUE ("Value (Signaling)")) -> ()  [unwired: 2 in, 2 out]
                                }
                                }
                                }
                                frame True {
                                n2492 = flat-sequence {
                                tunnel: w3711 -> [w3712]
                                frame #0 {
                                n2493 = property on="Trap Delta (MHz)" class="DigNum (strict)"("Val(Sgnl)"=w3712) -> ()  [unwired: 2 in, 2 out]
                                }
                                frame #1 {
                                n2494 = Wait (ms)(milliseconds to wait=u32 500) -> ()  [unwired: 1 out]
                                }
                                frame #2 {
                                n2495 = local read "Shift confocal"() -> (w3718:bool)
                                n2496 = local read "Mean"() -> (w3719:dbl)
                                n2497 = Greater?(x=w3719, y=11.0) -> (0:w3717:bool)
                                n2498 = And(x=w3717, y=w3718) -> (x .and. y?=w3715:bool)
                                n2499 = Not(x=w3717) -> (.not. x?=w3716:bool)
                                n2500 = And(x=w3716, y=w3718) -> (x .and. y?=w3714:bool)
                                n2501 = case shown="True" w3715 {
                                frame False {
                                }
                                frame True {
                                n2502 = local read "Confocal Y 2 (V)"() -> (w3724:dbl)